vi "Read Online Data.vi"(8 "Error In":errorcluster, 10 "Metodo de Entrada":T3(ring), 11 "Config Out":T1={"_RAW_ Traces"=[{"Trace Name"="V(vcc)", "Trace Type"="voltage", "Trace Raw Data"=array[50020 elements], "Trace Waveform"={"t0"=timestamp(0 s since 1904-01-01), "dt"=9.996001599360256e-07, "Y"=array[50020 elements]}}, {"Trace Name"="V(out+)", "Trace Type"="voltage", "Trace Raw Data"=array[50020 elements], "Trace Waveform"={"t0"=timestamp(0 s since 1904-01-01), "dt"=9.996001599360256e-07, "Y"=array[50020 elements]}}, {"Trace Name"="V(n004)", "Trace Type"="voltage", "Trace Raw Data"=array[50020 elements], "Trace Waveform"={"t0"=timestamp(0 s since 1904-01-01), "dt"=9.996001599360256e-07, "Y"=array[50020 elements]}}, {"Trace Name"="V(n001)", "Trace Type"="voltage", "Trace Raw Data"=array[50020 elements], "Trace Waveform"={"t0"=timestamp(0 s since 1904-01-01), "dt"=9.996001599360256e-07, "Y"=array[50020 elements]}}, {"Trace Name"="V(n002)", "Trace Type"="voltage", "Trace Raw Data"=array[50020 elements], "Trace Waveform"={"t0"=timestamp(0 s since 1904-01-01), "dt"=9.996001599360256e-07, "Y"=array[50020 elements]}}, {"Trace Name"="V(n003)", "Trace Type"="voltage", "Trace Raw Data"=array[50020 elements], "Trace Waveform"={"t0"=timestamp(0 s since 1904-01-01), "dt"=9.996001599360256e-07, "Y"=array[50020 elements]}}, {"Trace Name"="I(C2)", "Trace Type"="device_current", "Trace Raw Data"=array[50020 elements], "Trace Waveform"={"t0"=timestamp(0 s since 1904-01-01), "dt"=9.996001599360256e-07, "Y"=array[50020 elements]}}, {"Trace Name"="I(C1)", "Trace Type"="device_current", "Trace Raw Data"=array[50020 elements], "Trace Waveform"={"t0"=timestamp(0 s since 1904-01-01), "dt"=9.996001599360256e-07, "Y"=array[50020 elements]}}, {"Trace Name"="I(R3)", "Trace Type"="device_current", "Trace Raw Data"=array[50020 elements], "Trace Waveform"={"t0"=timestamp(0 s since 1904-01-01), "dt"=9.996001599360256e-07, "Y"=array[50020 elements]}}, {"Trace Name"="I(R2)", "Trace Type"="device_current", "Trace Raw Data"=array[50020 elements], "Trace Waveform"={"t0"=timestamp(0 s since 1904-01-01), "dt"=9.996001599360256e-07, "Y"=array[50020 elements]}}, {"Trace Name"="I(R1)", "Trace Type"="device_current", "Trace Raw Data"=array[50020 elements], "Trace Waveform"={"t0"=timestamp(0 s since 1904-01-01), "dt"=9.996001599360256e-07, "Y"=array[50020 elements]}}, {"Trace Name"="I(G1)", "Trace Type"="device_current", "Trace Raw Data"=array[50020 elements], "Trace Waveform"={"t0"=timestamp(0 s since 1904-01-01), "dt"=9.996001599360256e-07, "Y"=array[50020 elements]}}, {"Trace Name"="I(V3)", "Trace Type"="device_current", "Trace Raw Data"=array[50020 elements], "Trace Waveform"={"t0"=timestamp(0 s since 1904-01-01), "dt"=9.996001599360256e-07, "Y"=array[50020 elements]}}, {"Trace Name"="I(V2)", "Trace Type"="device_current", "Trace Raw Data"=array[50020 elements], "Trace Waveform"={"t0"=timestamp(0 s since 1904-01-01), "dt"=9.996001599360256e-07, "Y"=array[50020 elements]}}, {"Trace Name"="I(V1)", "Trace Type"="device_current", "Trace Raw Data"=array[50020 elements], "Trace Waveform"={"t0"=timestamp(0 s since 1904-01-01), "dt"=9.996001599360256e-07, "Y"=array[50020 elements]}}], "_WAV_ Traces"=[], "_MIC_ Config"={"task ID"=3, "Data Chunk Size"=0, "Num Channels"=0, "Resolution"=0, "Sampling Frequency"=0.0, "device ID"=0, "Num Chunks"=0}, "_LVM_ Traces"=[]} {"_MIC_ Config"."task ID" format="%.0x"}) -> (0 "Error Out":errorcluster, 1 "Channel 1":waveform(dbl), 2 "Channel 0":waveform(dbl))   [LabVIEW 2017, in "Aquisicao de Dados.lvlib"]
uses:
  Aquisicao de Dados.lvlib
  _ACC_DATA_ Config DAta State.ctl
  <vilib>/sound2/lvsound2.llb/Sound Input Task ID.ctl
  <vilib>/sound2/lvsound2.llb/Sound Data Format.ctl
  <vilib>/sound2/lvsound2.llb/Sampling Mode.ctl
  <vilib>/sound2/lvsound2.llb/Sound Input Read (DBL).vi
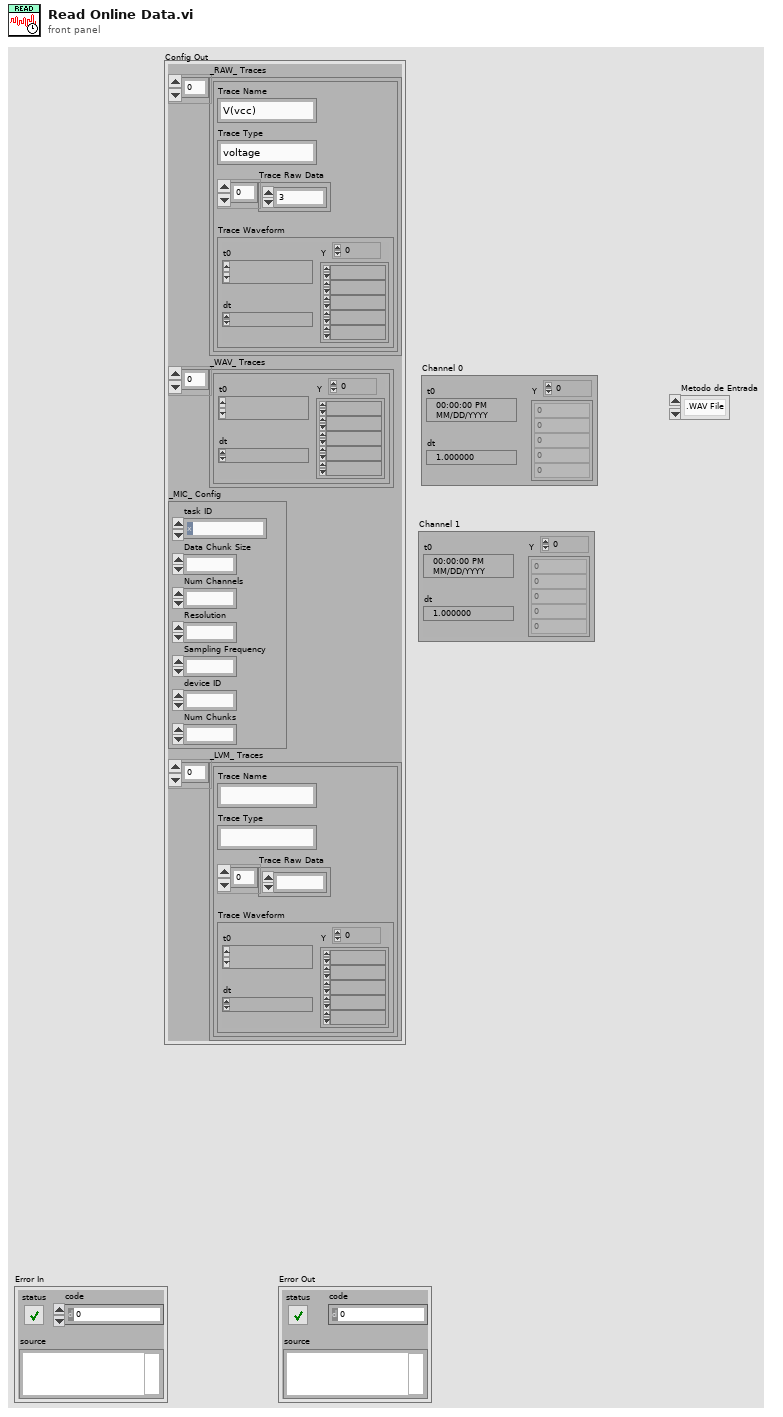
[diagram p1: front panel]
types:
  T1 = typedef "Aquisicao de Dados.lvlib/_ACC_DATA_ Config DAta State.ctl" = cluster{"_RAW_ Traces":cluster{"Trace Name":string, "Trace Type":string, "Trace Raw Data":dbl[], "Trace Waveform":waveform(dbl)}[], "_WAV_ Traces":waveform(dbl)[], "_MIC_ Config":cluster{"task ID":T2, "Data Chunk Size":i32, "Num Channels":i32, "Resolution":i32, "Sampling Frequency":dbl, "device ID":u32, "Num Chunks":i32}, "_LVM_ Traces":cluster{"Trace Name":string, "Trace Type":string, "Trace Raw Data":dbl[], "Trace Waveform":waveform(dbl)}[]}
  T2 = typedef "Sound Input Task ID.ctl" = u32
  T3 = enum32{".WAV File", "LTSpice Simulation", "Microphone", "MultiSim Simulation", "Serial Port"}
  T4 = cluster{"Trace Name":string, "Trace Type":string, "Trace Raw Data":dbl[], "Trace Waveform":waveform(dbl)}[]
  T5 = typedef "Sound Data Format.ctl" = cluster{"sample rate (S/s)":dbl, "number of channels":i32, "bits per sample":i32}
  T6 = cluster{"Trace Name":string, "Trace Type":string, "Trace Raw Data":dbl[], "Trace Waveform":waveform(dbl)}
  T7 = typedef "Sampling Mode.ctl" = i32
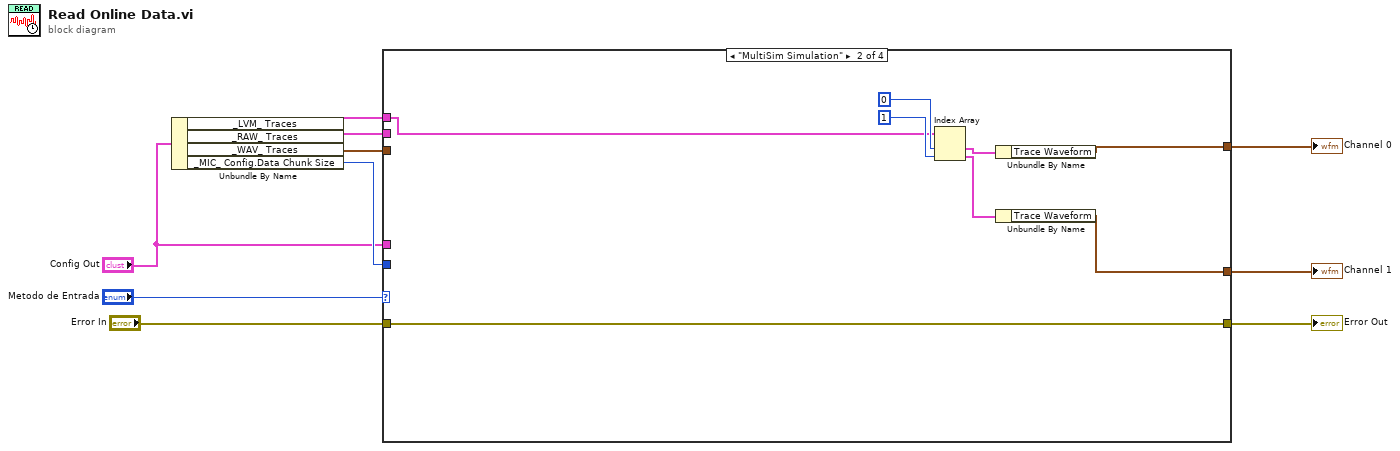
[diagram p0: block diagram]
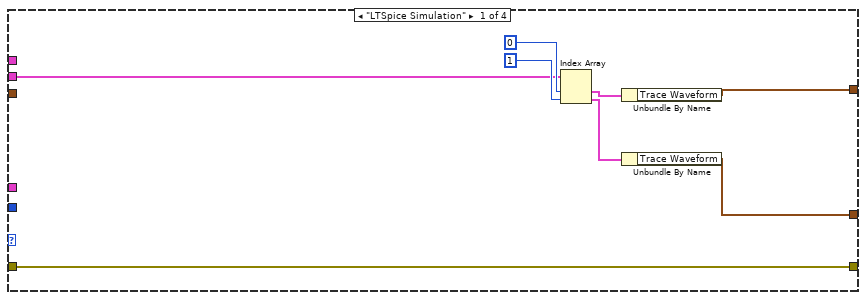
[diagram p2: hidden frame]
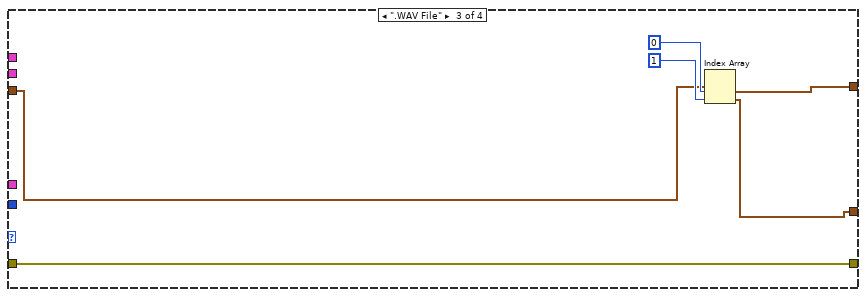
[diagram p3: hidden frame]
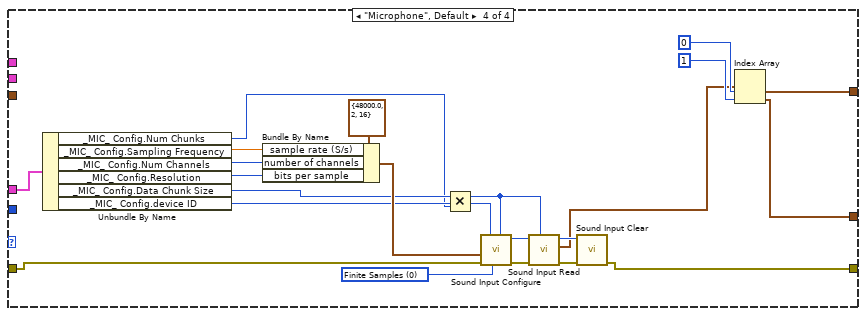
[diagram p4: hidden frame]
diagram:
  n1 = Unbundle By Name("Config Out") -> ("_LVM_ Traces"=w1:T4, "_RAW_ Traces"=w7:T4, "_WAV_ Traces"=w8:waveform(dbl)[], "_MIC_ Config.Data Chunk Size"=w9:i32)
  n2 = case shown="\"MultiSim Simulation\"" "Metodo de Entrada" {
    tunnel: "Error In" -> [w18 w26 w27 w39]
    tunnel: [w18 w26 w27 w37] -> w5
    tunnel: w8 -> [_ _ w28 _]
    tunnel: w7 -> [w15 _ _ _]
    tunnel: [w12 w21 w30 w51] -> w6
    tunnel: [w11 w20 w29 w52] -> w10
    tunnel: w9 -> [_ _ _ _]
    tunnel: "Config Out" -> [_ _ _ w38]
    tunnel: w1 -> [_ w19 _ _]
    frame "LTSpice Simulation" {
      n3 = Index Array(array=w15, index #1=0 ("index"), index #2=1 ("index")) -> (element #1=w14:T6, element #2=w13:T6)
      n4 = Unbundle By Name(w14) -> ("Trace Waveform"=w12:waveform(dbl))
      n5 = Unbundle By Name(w13) -> ("Trace Waveform"=w11:waveform(dbl))
    }
    frame "MultiSim Simulation" {
      n6 = Index Array(array=w19, index #1=0 ("index"), index #2=1 ("index")) -> (element #1=w23:T6, element #2=w22:T6)
      n7 = Unbundle By Name(w23) -> ("Trace Waveform"=w21:waveform(dbl))
      n8 = Unbundle By Name(w22) -> ("Trace Waveform"=w20:waveform(dbl))
    }
    frame ".WAV File" {
      n9 = Index Array(array=w28, index #1=0 ("index"), index #2=1 ("index")) -> (element #1=w30:waveform(dbl), element #2=w29:waveform(dbl))
    }
    frame "Microphone", Default {
      w45 = T7 0 items=["Finite Samples", "Continuous Samples"] ("sample mode")
      n10 = Unbundle By Name(w38) -> ("_MIC_ Config.Num Chunks"=w33:i32, "_MIC_ Config.Sampling Frequency"=w43:dbl, "_MIC_ Config.Num Channels"=w42:i32, "_MIC_ Config.Resolution"=w41:i32, "_MIC_ Config.Data Chunk Size"=w35:i32, "_MIC_ Config.device ID"=w40:u32)
      n11 = Bundle By Name(cluster=T5 {"sample rate (S/s)"=48000.0, "number of channels"=2, "bits per sample"=16} ("sound format"), "sample rate (S/s)"=w43, "number of channels"=w42, "bits per sample"=w41) -> (w44:T5)
      n12 = Multiply(x=w35, y=w33) -> (x*y=w34:i32)
      n13 = call <vilib>:"Sound Input Configure.vi"("number of samples/ch"=w34, "sample mode"=w45, "error in (no error)"=w39, "sound format"=w44, "device ID"=w40) -> ("error out"=w47:errorcluster, "task ID"=w46:T2)  [unwired: 5 in]
      n14 = call-poly <vilib>:"Sound Input Read.vi"("number of samples/ch"=w34, "error in (no error)"=w47, "task ID"=w46) -> ("error out"=w49:errorcluster, "data"=w36:waveform(dbl)[], "task ID out"=w48:T2)  [unwired: 6 in]
      n15 = call <vilib>:"Sound Input Clear.vi"("error in (no error)"=w49, "task ID"=w48) -> ("error out"=w37:errorcluster)  [unwired: 9 in]
      n16 = Index Array(array=w36, index #1=0 ("index"), index #2=1 ("index")) -> (element #1=w51:waveform(dbl), element #2=w52:waveform(dbl))
    }
  }
  "Channel 1" <- w10
  "Channel 0" <- w6
  "Error Out" <- w5
